vi "UHR-Fleezers Control (host) - 12.6.1.vi"() -> ()   [LabVIEW 2012] (continued)
        n1578 = Decrement(x=w2209) -> (x-1=w2210:u64)
        n1579 = Select(t=w2209, s=w2211, f=w2210) -> (s? t:f=w2208:u64)
        "Cycles/step (AOD)" <- w2208
        n1580 = xnode "Read/Write Control"("FPGA VI Reference In"=w2301, "error in"=w2300, "Scan steps"=w2240, "Number of scans"="Number of F/B Scans (AOD)", "Cycles per step"=w2208, "Scan freq.  increment"=w2246, "Scan BD"="Scan BD") -> ("error out"=w2299:errorcluster)  [unwired: 1 out]
        n1581 = Multiply(x=w2240, y=w2208) -> (x*y=w2294:u64)
        n1582 = Multiply(x=w2294, y=u64 2) -> (x*y=w2216:u64)
        n1583 = Multiply(x=w2217, y=w2216) -> (x*y=w2215:dbl)
        "Data points/scan (f/b)" <- w2215
        n1584 = Multiply(x=w2215, y="Number of F/B Scans (AOD)") -> (x*y=w2297:dbl)
        "Data points/scans" <- w2297
        n1585 = Divide(x=w2297, y=w2251) -> (x/y=→"N sets should be saved":dbl)
        n1586 = Multiply(x=w2294, y=w2235) -> (x*y=w2233:dbl)
        "Time/Scan (s) (AOD)" <- w2233
        n1587 = Select(t=w2265, s="Scan BD", f=0.0) -> (s? t:f=w2291:dbl)
        n1588 = Select(t=0.0, s="Scan BD", f=w2265) -> (s? t:f=w2287:dbl)
        n1589 = local read "BD 2 Frequency 2 (MHz)"() -> (w2283:dbl)
        n1590 = local read "BD 1 Frequency 2 (MHz)"() -> (w2286:dbl)
        n1591 = Add(x=w2287, y=w2258) -> (x+y=w2284:dbl)
        n1592 = Add(x=w2252, y=w2291) -> (x+y=w2285:dbl)
        n1593 = Multiply(x=w2233, y=2.0) -> (x*y=w2232:dbl)
        n1594 = Multiply(x=w2232, y="Number of F/B Scans (AOD)") -> (x*y=w2229:dbl)
        n1595 = Divide(x=w2229, y=60.0) -> (x/y=→"Time to Finish All (min)":dbl)
        n1596 = Add(x="Trap 2 Bead Size (nm)", y="Trap 1 Bead Size (nm)") -> (x+y=w2273:dbl)
        n1597 = Divide(x=w2273, y=2.0) -> (x/y=w2267:dbl)
        n1598 = local read "Initial delta (MHz)"() -> (w2270:dbl)
        n1599 = Subtract(x=w2284, y=w2283) -> (x-y=w2281:dbl)
        n1600 = Subtract(x=w2285, y=w2286) -> (x-y=w2282:dbl)
        n1601 = Square(x=w2281) -> (x^2=w2280:dbl)
        n1602 = Square(x=w2282) -> (x^2=w2279:dbl)
        n1603 = Add(x=w2279, y=w2280) -> (x+y=w2278:dbl)
        n1604 = Square Root(x=w2278) -> (sqrt(x)=w2277:dbl)
        "Final delta (MHz)" <- w2277
        n1605 = Multiply(x=w2269, y=w2277) -> (x*y=w2276:dbl)
        n1606 = Multiply(x=w2270, y=w2269) -> (x*y=w2268:dbl)
        n1607 = Subtract(x=w2268, y=w2267) -> (x-y=→"Initial sep (nm)":dbl)
        n1608 = Subtract(x=w2276, y=w2267) -> (x-y=→"Final sep (nm)":dbl)
      }
      event "Freq or Amp switch first", "Swap F1 and F2", "Freq switch delay", "Amp switch delay": Value Change {
        n1609 = event-data() -> ()  [unwired: 7 out]
        n1610 = local read "Amp switch delay"() -> (w2302:u16)
        n1611 = local read "Swap F1 and F2"() -> (w2303:bool)
        n1612 = xnode "Read/Write Control"("FPGA VI Reference In"=w2306, "error in"=w2305, "Swap F1 and F2"=w2303, "Amp switch delay"=w2302) -> ("error out"=w2304:errorcluster)  [unwired: 1 out]
      }
      event "Scan steps (MCL)", "Number of scans (MCL)", "Scan Range (V)\n(of steps)", "2D or 1D Scan", "N APD Samp/step", "Fast Scan Dir", "Continuous MCL Scanning", "Scan lines (y)": Value Change {
        w2308 = 32767.0 ("y")
        n1613 = event-data() -> ()  [unwired: 7 out]
        n1614 = Select(t="Scan lines (y)", s="2D or 1D Scan", f="Number of scans (MCL)") -> (s? t:f=w2313:u64)
        n1615 = Decrement(x="Scan steps (MCL)") -> (x-1=w2329:u64)
        n1616 = Divide(x="Scan Range (V)\n(of steps)", y=w2329) -> (x/y=w2328:dbl)
        "Desired Scan Incr (V)" <- w2328
        n1617 = local read "APD Integration Time (s)"() -> (w2321:dbl)
        n1618 = Multiply(x=w2328, y=w2308) -> (x*y=w2337:dbl)
        n1619 = Divide(x=w2337, y=10.0) -> (x/y=w2327:dbl)
        "Desired incr (int)" <- w2327
        n1620 = local read "Update Count (MCL)"() -> (w2333:u32)
        n1621 = Round Toward -Infinity(1:w2327) -> (0:w2336:dbl)
        n1622 = To Word Integer(number=w2336) -> (16bit integer=w2311:i16)
        "Actual Incr. int (MCL)" <- w2311
        n1623 = Multiply(x=w2321, y=40000000.0) -> (x*y=w2334:dbl)
        n1624 = Divide(x=w2334, y=w2333) -> (x/y=w2332:dbl)
        n1625 = Multiply(x=i16 10, y=w2311) -> (x*y=w2309:i16)
        n1626 = Multiply(x="N APD Samp/step", y=w2332) -> (x*y=w2331:dbl)
        "Cycles/step (MCL)" <- w2331
        n1627 = Divide(x=w2309, y=w2308) -> (x/y=→"Actual MCL Inc (V)":dbl)
        n1628 = Multiply(x="N APD Samp/step", y="Scan steps (MCL)") -> (x*y=w2323:dbl)
        n1629 = local read "APD Samples/FIFO Acq."() -> (w2320:dbl)
        n1630 = Multiply(x=w2323, y=u64 2) -> (x*y=w2322:dbl)
        "Data points/scan (f+b)" <- w2322
        n1631 = Multiply(x=w2322, y=w2313) -> (x*y=w2340:dbl)
        "Data points/scans (MCL)" <- w2340
        n1632 = Multiply(x=w2321, y=w2322) -> (x*y=w2314:dbl)
        "Time/f+b scan (s) (MCL)" <- w2314
        n1633 = Divide(x=w2340, y=w2320) -> (x/y=→"N sets should be saved (MCL)":dbl)
        n1634 = Multiply(x=w2314, y=w2313) -> (x*y=→"Total Time (s)":dbl)
        n1635 = Not(x="Fast Scan Dir") -> (.not. x?=w2318:bool)
        n1636 = xnode "Read/Write Control"("FPGA VI Reference In"=w2344, "error in"=w2343, "Scan steps (MCL)"="Scan steps (MCL)", "Number of scans (MCL)"=w2313, "Cycles per step (MCL)"=w2331, "Scan freq.  increment (MCL)"=w2311, "1D or 2D Scan?"="2D or 1D Scan", "MCL Scan Axis"=w2318, "Cont. Scan (MCL)"="Continuous MCL Scanning") -> ("error out"=w2342:errorcluster)  [unwired: 1 out]
      }
      event "Read Cal": Value Change {
        w2346 = 1000.0 ("y")
        n1637 = event-data() -> ()  [unwired: 7 out]
        n1638 = local read "Save file name"() -> (w2371:path)
        n1639 = local write "Read Cal"(FALSE ("Read Cal")) -> ()
        n1640 = Strip Path(path=w2371) -> (stripped path=w2370:path)  [unwired: 1 out]
        n1641 = Path To String(path=w2370) -> (string=w2369:string)
        n1642 = Concatenate Strings(w2369, "\\current.cal" ("string")) -> (w2367:string)
        n1643 = String To Path(string=w2367) -> (path=w2366:path)
        n1644 = Open/Create/Replace File(file path (use dialog)=w2366, operation (0:open)=T29."open", access (0:read/write)=enum16{"read/write", "read-only", "write-only"}."read-only") -> (refnum out=w2374:refnum<file>, error out=w2360:errorcluster)  [unwired: 1 in, 3 out]
        n1645 = Deny Access(4:w2360, 7:w2374) -> (0:w2359:errorcluster, 3:w2365:refnum<file>)  [unwired: 1 out]
        n1646 = Read from Binary File(5:0.0, 8:w2359, 9:T28."big-endian, network order" ("byte order (0:big-endian, network order)"), 10:-1 ("count (1)"), 11:w2365) -> (0:w2358:errorcluster, 2:w2356:dbl[], 3:w2361:refnum<file>)  [unwired: 2 out]
        n1647 = Array To Cluster(array=w2356) -> (cluster=w2355:T31)
        n1648 = Unbundle(w2355) -> ("[0]"=w2354:dbl, "[1]"=w2353:dbl, "[2]"=w2352:dbl, "[3]"=w2351:dbl, "[4]"=w2350:dbl, "[5]"=w2349:dbl)
        n1649 = Close File(refnum=w2361, error in=w2358) -> (error out=→"Read cal error":errorcluster)  [unwired: 1 out]
        n1650 = Multiply(x=w2349, y=w2346) -> (x*y=w2347:dbl)
        n1651 = local write "T2 kappa_x (pN/nm)"(w2351) -> ()
        n1652 = local write "T1 kappa_x (pN/nm)"(w2352) -> ()
        n1653 = local write "T1 alpha_x (nm/V)"(w2354) -> ()
        n1654 = local write "T2 alpha_x (nm/V)"(w2353) -> ()
        n1655 = Multiply(x=w2350, y=w2346) -> (x*y=w2348:dbl)
        n1656 = local write "T1 offset_x (mV)"(w2348) -> ()
        n1657 = local write "T2 offset_x (mV)"(w2347) -> ()
      }
      event "Abort MCL Scan": Value Change {
        n1658 = event-data() -> ()  [unwired: 7 out]
        n1659 = local write "MCL Scanning"(FALSE ("MCL Scanning")) -> ()
        n1660 = xnode "Read/Write Control"("FPGA VI Reference In"=w2379, "error in"=w2378, "Abort scan (MCL)"="Abort MCL Scan") -> ("error out"=w2377:errorcluster)  [unwired: 1 out]
      }
      event "Update Count (MCL)": Value Change {
        n1661 = event-data() -> ()  [unwired: 7 out]
        n1662 = xnode "Read/Write Control"("FPGA VI Reference In"=w2383, "error in"=w2382, "MCL count"="Update Count (MCL)") -> ("error out"=w2381:errorcluster)  [unwired: 1 out]
      }
      event "+ phase (MCL)", "- phase (MCL)": Value Change {
        n1663 = event-data() -> ()  [unwired: 7 out]
        n1664 = Or(x="- phase (MCL)", y="+ phase (MCL)") -> (x .or. y?=w2386:bool)
        n1665 = Negate(x="Phase adjust (MCL)") -> (-x=w2392:i16)
        n1666 = Select(t=w2392, s="+ phase (MCL)", f="Phase adjust (MCL)") -> (s? t:f=w2390:i16)
        n1667 = xnode "Read/Write Control"("FPGA VI Reference In"=w2394, "error in"=w2393, "Phase count adjustment (MCL)"=w2390) -> ("FPGA VI Reference Out"=w2387:T20, "error out"=w2388:errorcluster)
        n1668 = xnode "Read/Write Control"("FPGA VI Reference In"=w2387, "error in"=w2388, "+ phase (MCL)"=w2386) -> ("error out"=w2385:errorcluster)  [unwired: 1 out]
      }
      event "Abort AOD Scan": Value Change {
        n1669 = event-data() -> ()  [unwired: 7 out]
        n1670 = xnode "Read/Write Control"("FPGA VI Reference In"=w2398, "error in"=w2397, "Abort scan"="Abort AOD Scan") -> ("error out"=w2396:errorcluster)  [unwired: 1 out]
      }
      event "Continuous AOD Scanning": Value Change {
        n1671 = event-data() -> ()  [unwired: 7 out]
        n1672 = xnode "Read/Write Control"("FPGA VI Reference In"=w2402, "error in"=w2401, "Cont. Scan"="Continuous AOD Scanning") -> ("error out"=w2400:errorcluster)  [unwired: 1 out]
      }
      event "Index": Value Change {
        n1673 = event-data() -> ()  [unwired: 7 out]
        n1674 = call "Create new save file.vi"("Insert"="", "Ext"=".dat" ("string"), "Index In"="Index") -> ("Path Out"=→"Save file name":path, "Index Out"=w2403:dbl)
        "Save index" <- w2403
        n1675 = local write "Index"(w2403) -> ()
      }
      event "AO1", "AO2": Value Change {
        w2418 = 10.0 ("y")
        w2417 = 32767.0 ("y")
        n1676 = event-data() -> ()  [unwired: 7 out]
        n1677 = local read "AO2"() -> (w2416:dbl)
        n1678 = local read "AO1"() -> (w2413:dbl)
        n1679 = Multiply(x=w2413, y=w2417) -> (x*y=w2412:dbl)
        n1680 = Multiply(x=w2416, y=w2417) -> (x*y=w2415:dbl)
        n1681 = Divide(x=w2412, y=w2418) -> (x/y=w2411:dbl)
        n1682 = Divide(x=w2415, y=w2418) -> (x/y=w2414:dbl)
        n1683 = To Word Integer(number=w2411) -> (16bit integer=w2419:i16)
        n1684 = To Word Integer(number=w2414) -> (16bit integer=w2420:i16)
        n1685 = xnode "Read/Write Control"("FPGA VI Reference In"=w2410, "error in"=w2409, "AO1"=w2419, "AO2"=w2420) -> ("error out"=w2408:errorcluster)  [unwired: 1 out]
      }
      event "Inject Pump 1": Value Change {
        n1686 = event-data() -> ()  [unwired: 7 out]
        n1687 = local read "Use Harvard pumps\nfor beads (else Chemyx)"() -> (w2422:bool)
        n1688 = case shown="True" w2422 {
          tunnel: "Inject Pump 1" -> [w2426 w2464]
          tunnel: w2421 -> [_ w2465]
          frame False {
            n1689 = local read "Pump write delay (ms)"() -> (w2425:dbl)
            n1690 = local read "Chemyx Syringe Pump Serial Port"() -> (w2424:refnum<visa-resource-name>)
            n1691 = case shown="True" w2426 {
              tunnel: w2425 -> [w2432 w2446]
              tunnel: w2424 -> [w2429 w2445]
              frame False {
                n1692 = flat-sequence {
                  tunnel: w2429 -> [w2433]
                  tunnel: [w2433] -> w2430
                  tunnel: w2432 -> [_]
                  tunnel: [w2436] -> w2431
                  tunnel: w2430 -> [w2436]
                  tunnel: w2431 -> [w2437]
                  tunnel: [w2437] -> w2427
                  tunnel: [w2439] -> w2428
                  tunnel: w2427 -> [w2439]
                  tunnel: w2428 -> [w2441]
                  frame #0 {
                    n1693 = call "Write to pump.vi"("string"="enter pump1", "VISA resource name"=w2433) -> ()  [unwired: 1 out]
                  }
                  frame #1 {
                    n1694 = Wait (ms)(milliseconds to wait="Pump pause delay (ms)") -> ()  [unwired: 1 out]
                  }
                  frame #2 {
                    n1695 = call "Write to pump.vi"("string"="stop", "VISA resource name"=w2437) -> ()  [unwired: 1 out]
                  }
                  frame #3 {
                    n1696 = Wait (ms)(milliseconds to wait=u32 500) -> ()  [unwired: 1 out]
                  }
                  frame #4 {
                    n1697 = call "Write to pump.vi"("string"="stop", "VISA resource name"=w2441) -> ()  [unwired: 1 out]
                  }
                }
              }
              frame True {
                n1698 = flat-sequence {
                  tunnel: w2445 -> [w2455]
                  tunnel: w2446 -> [w2450]
                  tunnel: w2446 -> [w2457]
                  tunnel: w2445 -> [w2458]
                  tunnel: [w2458] -> w2443
                  tunnel: [w2460] -> w2444
                  tunnel: w2443 -> [w2460]
                  tunnel: w2444 -> [w2462]
                  frame #0 {
                    n1699 = local read "All Pump Parameters"() -> (w2449:T5)
                    n1700 = Unbundle By Name(w2449) -> ("Pump 1"=w2456:T32)
                    n1701 = call "Set pump parameters.vi"("Pump write delay (ms)"=w2450, "Volume (uL)"="Ch 1 Inject Volume (uL)", "Rate (uL/h)"="Ch 1 Inject Rate (ul/h)", "Units"=4.0, "Pump #"=1.0, "Pump Parameters In"=w2456, "VISA resource name"=w2455) -> ("Pump Parameters Out"=w2448:T32)  [unwired: 3 in]
                    n1702 = Bundle By Name(cluster=w2449, "Pump 1"=w2448) -> (w2447:T5)
                    n1703 = local write "All Pump Parameters"(w2447) -> ()
                  }
                  frame #1 {
                    n1704 = Wait (ms)(milliseconds to wait=w2457) -> ()  [unwired: 1 out]
                  }
                  frame #2 {
                    n1705 = call "Write to pump.vi"("string"="start", "VISA resource name"=w2458) -> ()  [unwired: 1 out]
                  }
                  frame #3 {
                    n1706 = Wait (ms)(milliseconds to wait=u32 500) -> ()  [unwired: 1 out]
                  }
                  frame #4 {
                    n1707 = call "Write to pump.vi"("string"="start", "VISA resource name"=w2462) -> ()  [unwired: 1 out]
                  }
                }
              }
            }
          }
          frame True {
            n1708 = case shown="False" w2464 {
              tunnel: w2465 -> [w2466 w2476]
              frame False {
                n1709 = flat-sequence {
                  tunnel: w2466 -> [w2468]
                  frame #0 {
                    n1710 = local write "Flushing P1"(FALSE ("Flushing P1")) -> ()
                    n1711 = Concatenate Strings("stop" ("string"), "\r") -> (w2470:string)
                    n1712 = VISA Write(VISA resource name=w2468, write buffer=w2470) -> ()  [unwired: 1 in, 3 out]
                  }
                  frame #1 {
                    n1713 = property on="Clear Volume P1" class="Bool (strict)"("Val(Sgnl)"=TRUE ("Value (Signaling)")) -> ()  [unwired: 2 in, 2 out]
                  }
                }
              }
              frame True {
                n1714 = local read "Normal Flow Rate (ul/h) P1"() -> (w2474:dbl)
                n1715 = Number To Decimal String(number=w2474) -> (decimal integer string=w2480:string)  [unwired: 1 in]
                n1716 = Concatenate Strings("irate  " ("string"), w2480, " u/h" ("string"), "\r") -> (w2478:string)
                n1717 = VISA Write(VISA resource name=w2476, write buffer=w2478) -> (VISA resource name out=w2475:refnum<visa-resource-name>)  [unwired: 1 in, 2 out]
                n1718 = Concatenate Strings("irun" ("string"), "\r") -> (w2482:string)
                n1719 = VISA Write(VISA resource name=w2475, write buffer=w2482) -> ()  [unwired: 1 in, 3 out]
              }
            }
          }
        }
      }
      event "Inject Pump 3": Value Change {
        n1720 = event-data() -> ()  [unwired: 7 out]
        n1721 = local read "Use Harvard pumps\nfor beads (else Chemyx)"() -> (w2485:bool)
        n1722 = case shown="True" w2485 {
          tunnel: "Inject Pump 3" -> [w2489 w2528]
          tunnel: w2484 -> [_ w2527]
          frame False {
            n1723 = local read "Pump write delay (ms)"() -> (w2488:dbl)
            n1724 = case shown="True" w2489 {
              tunnel: w2488 -> [w2495 w2509]
              tunnel: "Chemyx Syringe Pump Serial Port" -> [w2492 w2508]
              frame False {
                n1725 = flat-sequence {
                  tunnel: w2492 -> [w2496]
                  tunnel: [w2496] -> w2493
                  tunnel: w2495 -> [_]
                  tunnel: [w2499] -> w2494
                  tunnel: w2493 -> [w2499]
                  tunnel: w2494 -> [w2500]
                  tunnel: [w2500] -> w2490
                  tunnel: [w2502] -> w2491
                  tunnel: w2490 -> [w2502]
                  tunnel: w2491 -> [w2504]
                  frame #0 {
                    n1726 = call "Write to pump.vi"("string"="enter pump3", "VISA resource name"=w2496) -> ()  [unwired: 1 out]
                  }
                  frame #1 {
                    n1727 = local read "Pump pause delay (ms)"() -> (w2498:u32)
                    n1728 = Wait (ms)(milliseconds to wait=w2498) -> ()  [unwired: 1 out]
                  }
                  frame #2 {
                    n1729 = call "Write to pump.vi"("string"="stop", "VISA resource name"=w2500) -> ()  [unwired: 1 out]
                  }
                  frame #3 {
                    n1730 = Wait (ms)(milliseconds to wait=u32 0) -> ()  [unwired: 1 out]
                  }
                  frame #4 {
                    n1731 = call "Write to pump.vi"("string"="stop", "VISA resource name"=w2504) -> ()  [unwired: 1 out]
                  }
                }
              }
              frame True {
                n1732 = flat-sequence {
                  tunnel: w2508 -> [w2518]
                  tunnel: w2509 -> [w2513]
                  tunnel: w2509 -> [w2520]
                  tunnel: w2508 -> [w2521]
                  tunnel: [w2521] -> w2507
                  tunnel: [w2524] -> w2506
                  tunnel: w2507 -> [w2524]
                  tunnel: w2506 -> [w2525]
                  frame #0 {
                    n1733 = local read "All Pump Parameters"() -> (w2512:T5)
                    n1734 = Unbundle By Name(w2512) -> ("Pump 3"=w2519:T32)
                    n1735 = call "Set pump parameters.vi"("Pump write delay (ms)"=w2513, "Volume (uL)"="Ch 3 Inject Volume (uL)", "Rate (uL/h)"="Ch 3 Inject Rate (ul/h)", "Units"=4.0, "Pump #"=3.0, "Pump Parameters In"=w2519, "VISA resource name"=w2518) -> ("Pump Parameters Out"=w2511:T32)  [unwired: 3 in]
                    n1736 = Bundle By Name(cluster=w2512, "Pump 3"=w2511) -> (w2510:T5)
                    n1737 = local write "All Pump Parameters"(w2510) -> ()
                  }
                  frame #1 {
                    n1738 = Wait (ms)(milliseconds to wait=w2520) -> ()  [unwired: 1 out]
                  }
                  frame #2 {
                    n1739 = call "Write to pump.vi"("string"="start", "VISA resource name"=w2521) -> ()  [unwired: 1 out]
                  }
                  frame #3 {
                    n1740 = Wait (ms)(milliseconds to wait=u32 500) -> ()  [unwired: 1 out]
                  }
                  frame #4 {
                    n1741 = call "Write to pump.vi"("string"="start", "VISA resource name"=w2525) -> ()  [unwired: 1 out]
                  }
                }
              }
            }
          }
          frame True {
            n1742 = case shown="False" w2528 {
              tunnel: w2527 -> [w2529 w2536]
              frame False {
                n1743 = flat-sequence {
                  tunnel: w2529 -> [w2531]
                  frame #0 {
                    n1744 = local write "Flushing P3"(FALSE ("Flushing P3")) -> ()
                    n1745 = Concatenate Strings("stop" ("string"), "\r") -> (w2533:string)
                    n1746 = VISA Write(VISA resource name=w2531, write buffer=w2533) -> ()  [unwired: 1 in, 3 out]
                  }
                  frame #1 {
                    n1747 = property on="Clear Volume P3" class="Bool (strict)"("Val(Sgnl)"=TRUE ("Value (Signaling)")) -> ()  [unwired: 2 in, 2 out]
                  }
                }
              }
              frame True {
                n1748 = local read "Normal Flow Rate (ul/h) P3"() -> (w2537:dbl)
                n1749 = Number To Decimal String(number=w2537) -> (decimal integer string=w2543:string)  [unwired: 1 in]
                n1750 = Concatenate Strings("irate  " ("string"), w2543, " u/h" ("string"), "\r") -> (w2541:string)
                n1751 = VISA Write(VISA resource name=w2536, write buffer=w2541) -> (VISA resource name out=w2539:refnum<visa-resource-name>)  [unwired: 1 in, 2 out]
                n1752 = Concatenate Strings("irun" ("string"), "\r") -> (w2545:string)
                n1753 = VISA Write(VISA resource name=w2539, write buffer=w2545) -> ()  [unwired: 1 in, 3 out]
              }
            }
          }
        }
      }
      event "Inject Pump 2": Value Change {
        n1754 = event-data() -> ()  [unwired: 7 out]
        n1755 = local read "Pump write delay (ms)"() -> (w2549:dbl)
        n1756 = flat-sequence {
          tunnel: w2547 -> [w2562]
          tunnel: w2549 -> [w2558]
          tunnel: "Inject Pump 2" -> [_]
          tunnel: w2549 -> [w2564]
          tunnel: w2547 -> [w2565]
          frame #0 {
            n1757 = local read "All Pump Parameters"() -> (w2557:T5)
            n1758 = Multiply(x=60.0, y="Flush Center Ch Rate (ul/m)") -> (x*y=w2554:dbl)
            n1759 = Unbundle By Name(w2557) -> ("Pump 2"=w2563:T32)
            n1760 = call "Set pump parameters.vi"("Pump write delay (ms)"=w2558, "Volume (uL)"="Flush Center Ch Volume (uL)", "Rate (uL/h)"=w2554, "Units"=3.0, "Pump #"=2.0, "Pump Parameters In"=w2563, "VISA resource name"=w2562) -> ("Pump Parameters Out"=w2556:T32)  [unwired: 3 in]
            n1761 = Bundle By Name(cluster=w2557, "Pump 2"=w2556) -> (w2555:T5)
            n1762 = local write "All Pump Parameters"(w2555) -> ()
            n1763 = Add(x="Flush Center Ch Volume (uL)", y="Total Volume\nFlushed (uL)") -> (x+y=w2551:dbl)
            n1764 = local write "Total Volume\nFlushed (uL)"(w2551) -> ()
          }
          frame #1 {
            n1765 = Wait (ms)(milliseconds to wait=w2564) -> ()  [unwired: 1 out]
          }
          frame #2 {
            n1766 = call "Write to pump.vi"("string"="start", "VISA resource name"=w2565) -> ()  [unwired: 1 out]
          }
        }
        n1767 = local read "Chemyx Syringe Pump Serial Port"() -> (w2547:refnum<visa-resource-name>)
      }
      event "Sample Channel\nFlow": Value Change {
        n1768 = event-data() -> ()  [unwired: 7 out]
        n1769 = Select(t="irun" ("string"), s="Sample Channel\nFlow", f="stop" ("string")) -> (s? t:f=w2569:string)
        n1770 = Concatenate Strings(w2569, "\r") -> (w2572:string)
        n1771 = VISA Write(VISA resource name=w2567, write buffer=w2572) -> ()  [unwired: 1 in, 3 out]
      }
      event "Start Flow": Value Change {
        n1772 = event-data() -> ()  [unwired: 7 out]
        n1773 = local write "Sample Channel\nFlow"(TRUE ("Sample Channel\nFlow")) -> ()
        n1774 = local write "Start Flow"(FALSE ("Start Flow")) -> ()
        n1775 = Concatenate Strings("irun" ("string"), "\r") -> (w2578:string)
        n1776 = VISA Write(VISA resource name=w2574, write buffer=w2578) -> ()  [unwired: 1 in, 3 out]
      }
      event "Stop Flow": Value Change {
        w2580 = FALSE ("Stop Flow")
        n1777 = event-data() -> ()  [unwired: 7 out]
        n1778 = local write "Stop Flow"(w2580) -> ()
        n1779 = local write "Sample Channel\nFlow"(w2580) -> ()
        n1780 = Concatenate Strings("stop" ("string"), "\r") -> (w2583:string)
        n1781 = VISA Write(VISA resource name=w2581, write buffer=w2583) -> ()  [unwired: 1 in, 3 out]
      }
      event "Flow rate (uL/h)": Value Change {
        n1782 = event-data() -> ()  [unwired: 7 out]
        n1783 = Number To Decimal String(number="Flow rate (uL/h)") -> (decimal integer string=w2590:string)  [unwired: 1 in]
        n1784 = Concatenate Strings("irate  " ("string"), w2590, " u/h" ("string"), "\r") -> (w2589:string)
        n1785 = VISA Write(VISA resource name=w2586, write buffer=w2589) -> ()  [unwired: 1 in, 3 out]
      }
      event "Flush Sample": Value Change {
        n1786 = event-data() -> ()  [unwired: 7 out]
        n1787 = flat-sequence {
          tunnel: w2595 -> [w2623]
          tunnel: [w2603] -> w2594
          tunnel: [w2597] -> w2592
          tunnel: w2594 -> [w2627]
          tunnel: [w2627] -> w2593
          tunnel: w2592 -> [w2626]
          tunnel: w2593 -> [w2632]
          frame #0 {
            # "set paramaters (rate, volume) for flush, clear volume"
            n1788 = Number To Decimal String(number="Flush rate (uL/m)") -> (decimal integer string=w2619:string)  [unwired: 1 in]
            n1789 = Concatenate Strings("irate  " ("string"), w2619, " u/m" ("string"), "\r") -> (w2621:string)
            n1790 = VISA Write(VISA resource name=w2623, write buffer=w2621) -> (VISA resource name out=w2617:refnum<visa-resource-name>)  [unwired: 1 in, 2 out]
            n1791 = Reciprocal(x="Flush rate (uL/m)") -> (1/x=w2600:dbl)
            n1792 = Number To Decimal String(number="Volume (uL)") -> (decimal integer string=w2608:string)  [unwired: 1 in]
            n1793 = Multiply(x="Volume (uL)", y=w2600) -> (x*y=w2599:dbl)
            n1794 = Concatenate Strings("tvolume  " ("string"), w2608, " u" ("string"), "\r") -> (w2606:string)
            n1795 = Multiply(x=w2599, y=60000.0) -> (x*y=w2597:dbl)
            n1796 = VISA Write(VISA resource name=w2617, write buffer=w2606) -> (VISA resource name out=w2605:refnum<visa-resource-name>)  [unwired: 1 in, 2 out]
            n1797 = Concatenate Strings("cvolume" ("string"), "\r") -> (w2604:string)
            n1798 = VISA Write(VISA resource name=w2605, write buffer=w2604) -> (VISA resource name out=w2615:refnum<visa-resource-name>)  [unwired: 1 in, 2 out]
            n1799 = Concatenate Strings("irun" ("string"), "\r") -> (w2613:string)
            n1800 = VISA Write(VISA resource name=w2615, write buffer=w2613) -> (VISA resource name out=w2603:refnum<visa-resource-name>)  [unwired: 1 in, 2 out]
          }
          frame #1 {
            # "Have to wait until\nflow is done to reset\nrate"
            n1801 = Add(x=w2626, y=100.0) -> (x+y=w2625:dbl)
            n1802 = Wait (ms)(milliseconds to wait=w2625) -> ()  [unwired: 1 out]
          }
          frame #2 {
            # "reset flow rate to usual flow rate"
            n1803 = local read "Flow rate (uL/h)"() -> (w2638:dbl)
            n1804 = Number To Decimal String(number=w2638) -> (decimal integer string=w2636:string)  [unwired: 1 in]
            n1805 = Concatenate Strings("irate  " ("string"), w2636, " u/h" ("string"), "\r") -> (w2634:string)
            n1806 = VISA Write(VISA resource name=w2632, write buffer=w2634) -> (VISA resource name out=w2628:refnum<visa-resource-name>)  [unwired: 1 in, 2 out]
            n1807 = Concatenate Strings("cvolume" ("string"), "\r") -> (w2629:string)
            n1808 = VISA Write(VISA resource name=w2628, write buffer=w2629) -> ()  [unwired: 1 in, 3 out]
          }
        }
      }
      event "Flush Pump 3": Value Change {
        n1809 = event-data() -> ()  [unwired: 7 out]
        n1810 = flat-sequence {
          tunnel: w2639 -> [w2642]
          frame #0 {
            # "set paramaters (rate, volume) for flush, clear volume"
            n1811 = Number To Decimal String(number="Flush rate (uL/m) P3") -> (decimal integer string=w2664:string)  [unwired: 1 in]
            n1812 = local write "Inject Pump 3"(TRUE ("Inject Pump 3")) -> ()
            n1813 = Concatenate Strings("irate  " ("string"), w2664, " u/m" ("string"), "\r") -> (w2666:string)
            n1814 = VISA Write(VISA resource name=w2642, write buffer=w2666) -> (VISA resource name out=w2662:refnum<visa-resource-name>)  [unwired: 1 in, 2 out]
            n1815 = Reciprocal(x="Flush rate (uL/m) P3") -> (1/x=w2646:dbl)
            n1816 = Number To Decimal String(number="Volume (uL) P3") -> (decimal integer string=w2653:string)  [unwired: 1 in]
            n1817 = Multiply(x="Volume (uL) P3", y=w2646) -> (x*y=w2645:dbl)
            n1818 = Concatenate Strings("tvolume  " ("string"), w2653, " u" ("string"), "\r") -> (w2651:string)
            n1819 = Multiply(x=w2645, y=60.0) -> (x*y=→"HP3 Flush Time (s)":dbl)
            n1820 = VISA Write(VISA resource name=w2662, write buffer=w2651) -> (VISA resource name out=w2650:refnum<visa-resource-name>)  [unwired: 1 in, 2 out]
            n1821 = Concatenate Strings("cvolume" ("string"), "\r") -> (w2649:string)
            n1822 = VISA Write(VISA resource name=w2650, write buffer=w2649) -> (VISA resource name out=w2660:refnum<visa-resource-name>)  [unwired: 1 in, 2 out]
            n1823 = Concatenate Strings("irun" ("string"), "\r") -> (w2658:string)
            n1824 = VISA Write(VISA resource name=w2660, write buffer=w2658) -> ()  [unwired: 1 in, 3 out]
          }
          frame #1 {
            "Flushing P3" <- TRUE ("Flushing P3")
          }
        }
      }
      event "Flush Pump 1": Value Change {
        n1825 = event-data() -> ()  [unwired: 7 out]
        n1826 = flat-sequence {
          tunnel: [w2680] -> w2670
          tunnel: w2669 -> [w2673]
          tunnel: w2670 -> [_]
          frame #0 {
            # "set paramaters (rate, volume) for flush, clear volume"
            n1827 = local write "Inject Pump 1"(TRUE ("Inject Pump 1")) -> ()
            n1828 = Number To Decimal String(number="Flush rate (uL/m) P1") -> (decimal integer string=w2696:string)  [unwired: 1 in]
            n1829 = Concatenate Strings("irate  " ("string"), w2696, " u/m" ("string"), "\r") -> (w2698:string)
            n1830 = VISA Write(VISA resource name=w2673, write buffer=w2698) -> (VISA resource name out=w2694:refnum<visa-resource-name>)  [unwired: 1 in, 2 out]
            n1831 = Reciprocal(x="Flush rate (uL/m) P1") -> (1/x=w2677:dbl)
            n1832 = Number To Decimal String(number="Volume (uL) P1") -> (decimal integer string=w2685:string)  [unwired: 1 in]
            n1833 = Multiply(x="Volume (uL) P1", y=w2677) -> (x*y=w2676:dbl)
            n1834 = Concatenate Strings("tvolume  " ("string"), w2685, " u" ("string"), "\r") -> (w2683:string)
            n1835 = Multiply(x=w2676, y=60.0) -> (x*y=→"HP1 Flush Time (s)":dbl)
            n1836 = VISA Write(VISA resource name=w2694, write buffer=w2683) -> (VISA resource name out=w2682:refnum<visa-resource-name>)  [unwired: 1 in, 2 out]
            n1837 = Concatenate Strings("cvolume" ("string"), "\r") -> (w2681:string)
            n1838 = VISA Write(VISA resource name=w2682, write buffer=w2681) -> (VISA resource name out=w2692:refnum<visa-resource-name>)  [unwired: 1 in, 2 out]
            n1839 = Concatenate Strings("irun" ("string"), "\r") -> (w2690:string)
            n1840 = VISA Write(VISA resource name=w2692, write buffer=w2690) -> (VISA resource name out=w2680:refnum<visa-resource-name>)  [unwired: 1 in, 2 out]
          }
          frame #1 {
            "Flushing P1" <- TRUE ("Flushing P3")
          }
        }
      }
      event "Clear Volume": Value Change {
        n1841 = event-data() -> ()  [unwired: 7 out]
        n1842 = Concatenate Strings("cvolume" ("string"), "\r") -> (w2702:string)
        n1843 = VISA Write(VISA resource name=w2701, write buffer=w2702) -> ()  [unwired: 1 in, 3 out]
      }
      event "Clear Volume P3": Value Change {
        n1844 = event-data() -> ()  [unwired: 7 out]
        n1845 = Concatenate Strings("cvolume" ("string"), "\r") -> (w2708:string)
        n1846 = VISA Write(VISA resource name=w2707, write buffer=w2708) -> ()  [unwired: 1 in, 3 out]
        n1847 = local write "Clear Volume P3"(FALSE ("Clear Volume P3")) -> ()
      }
      event "Clear Volume P1": Value Change {
        n1848 = event-data() -> ()  [unwired: 7 out]
        n1849 = Concatenate Strings("cvolume" ("string"), "\r") -> (w2713:string)
        n1850 = local write "Clear Volume P1"(FALSE ("Clear Volume P1")) -> ()
        n1851 = VISA Write(VISA resource name=w2712, write buffer=w2713) -> ()  [unwired: 1 in, 3 out]
      }
      event "Display On P3": Value Change {
        n1852 = event-data() -> ()  [unwired: 7 out]
        n1853 = Select(t="dim 100", s="Display On P3", f="dim 0") -> (s? t:f=w2719:string)
        n1854 = Concatenate Strings(w2719, "\r") -> (w2721:string)
        n1855 = VISA Write(VISA resource name=w2716, write buffer=w2721) -> ()  [unwired: 1 in, 3 out]
      }
      event "Display On P1": Value Change {
        n1856 = event-data() -> ()  [unwired: 7 out]
        n1857 = Select(t="dim 100", s="Display On P1", f="dim 0") -> (s? t:f=w2726:string)
        n1858 = Concatenate Strings(w2726, "\r") -> (w2728:string)
        n1859 = VISA Write(VISA resource name=w2723, write buffer=w2728) -> ()  [unwired: 1 in, 3 out]
      }
      event "Retract Pump 3": Value Change {
        n1860 = event-data() -> ()  [unwired: 7 out]
        n1861 = local write "Retract Pump 3"(FALSE ("Retract Pump 3")) -> ()
        n1862 = case shown="True" "Retract Pump 3" {
          tunnel: w2730 -> [_ w2733]
          frame False {
          }
          frame True {
            n1863 = Number To Decimal String(number="Retract Rate (uL/m)") -> (decimal integer string=w2751:string)  [unwired: 1 in]
            n1864 = Concatenate Strings("wrate  " ("string"), w2751, " u/m" ("string"), "\r") -> (w2753:string)
            n1865 = VISA Write(VISA resource name=w2733, write buffer=w2753) -> (VISA resource name out=w2744:refnum<visa-resource-name>)  [unwired: 1 in, 2 out]
            n1866 = Number To Decimal String(number="Retract Vol 3 (uL)") -> (decimal integer string=w2746:string)  [unwired: 1 in]
            n1867 = Concatenate Strings("tvolume  " ("string"), w2746, " u" ("string"), "\r") -> (w2743:string)
            n1868 = VISA Write(VISA resource name=w2744, write buffer=w2743) -> (VISA resource name out=w2739:refnum<visa-resource-name>)  [unwired: 1 in, 2 out]
            n1869 = Concatenate Strings("cvolume" ("string"), "\r") -> (w2740:string)
            n1870 = VISA Write(VISA resource name=w2739, write buffer=w2740) -> (VISA resource name out=w2734:refnum<visa-resource-name>)  [unwired: 1 in, 2 out]
            n1871 = Concatenate Strings("wrun" ("string"), "\r") -> (w2735:string)
            n1872 = VISA Write(VISA resource name=w2734, write buffer=w2735) -> ()  [unwired: 1 in, 3 out]
          }
        }
      }
      event "Retract Pump 1": Value Change {
        n1873 = event-data() -> ()  [unwired: 7 out]
        n1874 = local write "Retract Pump 1"(FALSE ("Retract Pump 1")) -> ()
        n1875 = case shown="True" "Retract Pump 1" {
          tunnel: w2755 -> [_ w2760]
          frame False {
          }
          frame True {
            n1876 = local read "Retract Rate (uL/m)"() -> (w2758:dbl)
            n1877 = Number To Decimal String(number=w2758) -> (decimal integer string=w2776:string)  [unwired: 1 in]
            n1878 = Concatenate Strings("wrate  " ("string"), w2776, " u/m" ("string"), "\r") -> (w2778:string)
            n1879 = VISA Write(VISA resource name=w2760, write buffer=w2778) -> (VISA resource name out=w2770:refnum<visa-resource-name>)  [unwired: 1 in, 2 out]
            n1880 = Number To Decimal String(number="Retract Vol 1 (uL)") -> (decimal integer string=w2772:string)  [unwired: 1 in]
            n1881 = Concatenate Strings("tvolume  " ("string"), w2772, " u" ("string"), "\r") -> (w2769:string)
            n1882 = VISA Write(VISA resource name=w2770, write buffer=w2769) -> (VISA resource name out=w2766:refnum<visa-resource-name>)  [unwired: 1 in, 2 out]
            n1883 = Concatenate Strings("cvolume" ("string"), "\r") -> (w2767:string)
            n1884 = VISA Write(VISA resource name=w2766, write buffer=w2767) -> (VISA resource name out=w2761:refnum<visa-resource-name>)  [unwired: 1 in, 2 out]
            n1885 = Concatenate Strings("wrun" ("string"), "\r") -> (w2762:string)
            n1886 = VISA Write(VISA resource name=w2761, write buffer=w2762) -> ()  [unwired: 1 in, 3 out]
          }
        }
      }
      event "Flip Green Filter": Value Change {
        n1887 = event-data() -> ()  [unwired: 7 out]
        n1888 = Not(x="Flip Green Filter") -> (.not. x?=w2780:bool)
        n1889 = local write "Flip Green Filter"(w2780) -> ()
        n1890 = flat-sequence {
          tunnel: w2788 -> [w2793]
          tunnel: w2787 -> [w2792]
          tunnel: [w2790] -> w2785
          tunnel: [w2789] -> w2784
          tunnel: [w2795] -> w2783
          tunnel: w2785 -> [w2795]
          tunnel: [w2794] -> w2782
          tunnel: w2784 -> [w2794]
          tunnel: w2783 -> [w2799]
          tunnel: w2782 -> [w2798]
          tunnel: [w2797] -> w2786
          frame #0 {
            n1891 = xnode "Read/Write Control"("FPGA VI Reference In"=w2793, "error in"=w2792, "Green Filter Flipper"=TRUE) -> ("FPGA VI Reference Out"=w2790:T20, "error out"=w2789:errorcluster)
          }
          frame #1 {
            n1892 = Wait (ms)(milliseconds to wait=u32 100) -> ()  [unwired: 1 out]
          }
          frame #2 {
            n1893 = xnode "Read/Write Control"("FPGA VI Reference In"=w2799, "error in"=w2798, "Green Filter Flipper"=FALSE) -> ("error out"=w2797:errorcluster)  [unwired: 1 out]
          }
        }
      }
      event "Pump 1 contents", "Pump 3 contents": Value Change {
        n1894 = event-data() -> ()  [unwired: 7 out]
        n1895 = local read "Pump 1 contents"() -> (→"Pump 1 cont disp":string)
        n1896 = local read "Pump 3 contents"() -> (→"Pump 3 cont disp":string)
      }
      event "Reset Trap Pos. FB": Value Change {
        n1897 = event-data() -> ()  [unwired: 7 out]
        n1898 = xnode "Read/Write Control"("FPGA VI Reference In"=w2805, "error in"=w2804, "Trap Pos. FB Reset"="Reset Trap Pos. FB") -> ()  [unwired: 2 out]
      }
      event "Rem fb disp offset": Value Change {
        n1899 = event-data() -> ()  [unwired: 7 out]
        n1900 = local write "Rem fb disp offset"(FALSE ("Rem fb disp offset")) -> ()
        n1901 = local read "Mean T1 Position (nm)"() -> (w2807:dbl)
        n1902 = local read "FB Trap Pos Offset"() -> (w2808:dbl)
        n1903 = Subtract(x=w2808, y=w2807) -> (x-y=w2806:dbl)
        n1904 = local write "FB Trap Pos Offset"(w2806) -> ()
      }
      event "Threshold (nm)": Value Change {
        n1905 = event-data() -> ()  [unwired: 7 out]
        n1906 = flat-sequence {
          tunnel: w2812 -> [w2820]
          tunnel: w2811 -> [w2819]
          tunnel: [w2813] -> w2810
          tunnel: w2810 -> [w2826]
          frame #0 {
            n1907 = xnode "Read/Write Control"("FPGA VI Reference In"=w2820, "error in"=w2819) -> ("FPGA VI Reference Out"=w2816:T20, "error out"=w2815:errorcluster, "FPGA TTrig Thresh"=w2817:i64)
            n1908 = local read "Threshold stored (nm)"() -> (w2825:dbl)
            n1909 = local read "Threshold (nm)"() -> (w2813:dbl)
            n1910 = local read "AOM X Cal (nm/MHz)"() -> (w2823:dbl)
            n1911 = Subtract(x=w2813, y=w2825) -> (x-y=w2824:dbl)
            n1912 = Divide(x=w2824, y=w2823) -> (x/y=w2821:dbl)
            n1913 = call "IR AOM freq to word.vi"("Frequency In (MHz)"=w2821) -> ("Frequency Word Out (double)"=w2822:dbl)
            n1914 = To Quad Integer(1:w2822) -> (0:w2818:i64)
            n1915 = Add(x=w2817, y=w2818) -> (x+y=w2814:i64)
            n1916 = xnode "Read/Write Control"("FPGA VI Reference In"=w2816, "error in"=w2815, "FPGA TTrig Thresh"=w2814) -> ()  [unwired: 2 out]
          }
          frame #1 {
            "Threshold stored (nm)" <- w2826
          }
        }
      }
      event "FB Trig Integrate": Value Change {
        n1917 = event-data() -> ()  [unwired: 7 out]
        n1918 = local read "FB Trig Integrate"() -> (w2828:u32)
        n1919 = xnode "Read/Write Control"("FPGA VI Reference In"=w2830, "error in"=w2829, "FB Trig Integrate"=w2828) -> ("error out"=w2827:errorcluster)  [unwired: 1 out]
      }
      event "11": Value Change {
        n1920 = event-data() -> ()  [unwired: 7 out]
        n1921 = local read "11"() -> (w2831:bool)
        n1922 = case shown="True" w2831 {
          frame False {
          }
          frame True {
            n1923 = local read "Messages"() -> (w2833:string)
            n1924 = call "Update messages.vi"("Message to add"="You kicked it up to 11!", "Old message string"=w2833) -> ("New message string"=w2834:string)
            n1925 = call <vilib>:"Beep.vi"() -> ()  [unwired: 12 in]
            n1926 = local write "Messages"(w2834) -> ()
          }
        }
      }
      event "Trap Pos. FB ON": Value Change {
        n1927 = event-data() -> ()  [unwired: 7 out]
        n1928 = xnode "Read/Write Control"("FPGA VI Reference In"=w2837, "error in"=w2836, "Force feedback"="Trap Pos. FB ON") -> ()  [unwired: 2 out]
      }
      event "Remove Action Offset": Value Change {
        n1929 = event-data() -> ()  [unwired: 7 out]
        n1930 = local write "Remove Action Offset"(FALSE ("Remove Action Offset")) -> ()
        n1931 = local read "Trap Pos. FB Mult Factor"() -> (w2842:i64)
        n1932 = local read "Trap Pos FB Action"() -> (w2840:i64)
        n1933 = local read "Trap Pos. FB Offset Factor"() -> (w2838:i64)
        n1934 = Multiply(x=w2842, y=w2840) -> (x*y=w2841:i64)
        n1935 = Add(x=w2841, y=w2838) -> (x+y=w2839:i64)
        n1936 = local write "Trap Pos. FB Offset Factor"(w2839) -> ()
        n1937 = xnode "Read/Write Control"("FPGA VI Reference In"=w2845, "error in"=w2844, "Trap Pos. FB Offset Factor"=w2839) -> ()  [unwired: 2 out]
      }
      event "Remove Unwinding Offset": Value Change {
        n1938 = event-data() -> ()  [unwired: 7 out]
        n1939 = local write "Remove Unwinding Offset"(FALSE ("Remove Action Offset")) -> ()
        n1940 = local read "Trap Pos. FB Mult Factor"() -> (w2857:i64)
        n1941 = local read "Trap Pos FB Action"() -> (w2855:i64)
        n1942 = local read "Trap Pos. FB Offset Factor"() -> (w2854:i64)
        n1943 = Multiply(x=w2857, y=w2855) -> (x*y=w2856:i64)
        n1944 = local read "Trap Pos. FB Mult Factor"() -> (w2853:i64)
        n1945 = Add(x=w2856, y=w2854) -> (x+y=w2847:i64)
        n1946 = Multiply(x=32768, y="factor") -> (x*y=w2850:dbl)
        n1947 = Multiply(x=w2850, y=w2853) -> (x*y=w2852:dbl)
        n1948 = Subtract(x=w2847, y=w2852) -> (x-y=w2851:dbl)
        n1949 = To Quad Integer(1:w2851) -> (0:w2846:i64)
        n1950 = xnode "Read/Write Control"("FPGA VI Reference In"=w2860, "error in"=w2859, "Trap Pos. FB Offset Factor"=w2846) -> ()  [unwired: 2 out]
        n1951 = local write "Trap Pos. FB Offset Factor"(w2846) -> ()
      }
      event "Trap Pos. FB Range", "Trap Pos. FB Gains", "Trap Pos. FB Mult Factor", "Trap Pos. FB Offset Factor", "Trap Pos FB Negate Action", "Trap Pos FB Monitor\nT1 or T2", "Differential FB?", "Negate Diff?": Value Change {
        n1952 = event-data() -> ()  [unwired: 7 out]
        n1953 = Unbundle By Name("Trap Pos. FB Gains") -> ("proportional gain (Kc)"=w2863:fxp<+/-,16,8>, "integral gain (Kc*Ts/Ti)"=w2862:fxp<+/-,16,8>, "derivative gain (Kc*Td/Ts)"=w2861:fxp<+/-,16,8>)
        n1954 = local read "Negate Diff?"() -> (w2868:bool)
        n1955 = Unbundle By Name("Trap Pos. FB Range") -> ("output high"=w2866:fxp<+/-,16,1>, "output low"=w2865:fxp<+/-,16,1>)
        n1956 = xnode "Read/Write Control"("FPGA VI Reference In"=w2876, "error in"=w2875, "FB2 output high"=w2866, "FB2 output low"=w2865, "P2"=w2863, "I2"=w2862, "D2"=w2861, "Trap Pos. FB Mult Factor"="Trap Pos. FB Mult Factor", "Trap Pos. FB Offset Factor"="Trap Pos. FB Offset Factor", "Trap Pos FB Negate Action"="Trap Pos FB Negate Action", "Trap Pos FB Monitor T1 or T2"="Trap Pos FB Monitor\nT1 or T2", "AI1 X Scale"="Trap Pos. AI1 X Pre-scale", "Negate Diff?"=w2868, "Diff FB Measurement?"="Differential FB?") -> ()  [unwired: 2 out]
      }
      event "Trap Pos FB SP", "Trap Pos FB SP 2", "Use SP 2": Value Change {
        n1957 = event-data() -> ()  [unwired: 7 out]
        n1958 = Select(t="Trap Pos FB SP 2", s="Use SP 2", f="Trap Pos FB SP") -> (s? t:f=w2877:fxp<+/-,16,1>)
        n1959 = xnode "Read/Write Control"("FPGA VI Reference In"=w2882, "error in"=w2881, "Trap Pos. FB SP"=w2877) -> ()  [unwired: 2 out]
      }
      event "Offset SP2 from SP1": Value Change {
        n1960 = event-data() -> ()  [unwired: 7 out]
        n1961 = local read "Trap Pos FB SP"() -> (w2885:fxp<+/-,16,1>)
        n1962 = Add(x=w2885, y="SP2 Offset") -> (x+y=w2883:fxp<+/-,16,1>)
        n1963 = property on="Trap Pos FB SP 2" class="DigNum (strict)"("Val(Sgnl)"=w2883) -> ()  [unwired: 2 in, 2 out]
        n1964 = local write "Offset SP2 from SP1"(FALSE ("Offset SP2 from SP1")) -> ()
      }
      event "Set Reading to\nSetpoint": Value Change {
        # "This is the actual PID input signal"
        n1965 = event-data() -> ()  [unwired: 7 out]
        n1966 = local write "Set Reading to\nSetpoint"(FALSE ("Set SP to Reading")) -> ()
        n1967 = xnode "Read/Write Control"("FPGA VI Reference In"=w2891, "error in"=w2890) -> ("FPGA VI Reference Out"=w2889:T20, "error out"=w2888:errorcluster, "Trap Pos FB Int-Norm Signal"=w2887:fxp<+/-,16,1>)
        n1968 = local read "Differential FB?"() -> (w2892:bool)
        n1969 = case shown="False" w2892 {
          tunnel: [w2897 w2904] -> w2894
          tunnel: w2887 -> [w2895 w2904]
          frame False {
            n1970 = local read "Trap Pos FB Monitor\nT1 or T2"() -> (w2900:bool)
            n1971 = local read "Trap X AI1 (DMA)"() -> (w2903:T13)
            n1972 = Unbundle By Name(w2903) -> ("Set 1"=w2902:fxp<+/-,16,1>, "Set 2"=w2901:fxp<+/-,16,1>)
            n1973 = Select(t=w2902, s=w2900, f=w2901) -> (s? t:f=w2899:fxp<+/-,16,1>)
            n1974 = Not(x="Set SP Using...") -> (.not. x?=w2896:bool)
            n1975 = Select(t=w2895, s=w2896, f=w2899) -> (s? t:f=w2897:fxp<+/-,16,1>)
          }
          frame True {
          }
        }
        n1976 = xnode "Read/Write Control"("FPGA VI Reference In"=w2889, "error in"=w2888, "Trap Pos. FB SP"=w2894) -> ()  [unwired: 2 out]
        n1977 = local write "Trap Pos FB SP"(w2894) -> ()
      }
      event "Trap Pos. FB Out Scale 2^n": Value Change {
        n1978 = event-data() -> ()  [unwired: 7 out]
        n1979 = Scale By Power Of 2(n="Trap Pos. FB Out Scale 2^n", x=ext 1.0) -> (x*2^n=w2905:ext)
        n1980 = property on="Trap Pos. FB Mult Factor" class="DigNum (strict)"("Val(Sgnl)"=w2905) -> ()  [unwired: 2 in, 2 out]
      }
      event "Trap Pos FB Int Count": Value Change {
        n1981 = event-data() -> ()  [unwired: 7 out]
        n1982 = xnode "Read/Write Control"("FPGA VI Reference In"=w2910, "error in"=w2909, "Trap Pos FB Int Count"="Trap Pos FB Int Count") -> ()  [unwired: 2 out]
      }
      event "Trap pos": Value Change {
        n1983 = event-data() -> ()  [unwired: 7 out]
        n1984 = case shown="True" "Trap pos" {
          frame False {
            n1985 = property on="Trap Delta Graph" class="WFGraph (strict)"("Visible"=TRUE) -> ()  [unwired: 2 in, 2 out]
            n1986 = property on="Saved trap pos" class="WFGraph (strict)"("Visible"=FALSE) -> ()  [unwired: 2 in, 2 out]
          }
          frame True {
            n1987 = property on="Saved trap pos" class="WFGraph (strict)"("Visible"=TRUE) -> ()  [unwired: 2 in, 2 out]
            n1988 = property on="Trap Delta Graph" class="WFGraph (strict)"("Visible"=FALSE) -> ()  [unwired: 2 in, 2 out]
          }
        }
      }
    }
    "error out 2" <- w1733
    n1989 = node-c288() -> ()  [unwired: 2 out]
  }
  n1990 = while "Duncan's play event loop" {
    stop <- w2917 stop-if-true
    n1991 = Create User Event(user event datatype=TRUE ("Boolean")) -> (user event=w2918:refnum<user-event>)  [unwired: 1 in, 1 out]
    n1992 = Create User Event(user event datatype=TRUE ("Boolean")) -> (user event=w2925:refnum<user-event>)  [unwired: 1 in, 1 out]
    n1993 = global write "Global for fluorescence simulation mean (30 samples), (power series).vi" "Red Signal"(w2918) -> ()
    n1994 = global write "Global for fluorescence simulation mean (30 samples), (power series).vi" "Green Signal"(w2925) -> ()
    n1995 = register-events(w2925, w2918) -> (reference out=w2924:refnum<event-registration>)  [unwired: 2 in, 1 out]
    n1996 = event shown="[1] \"Get Fluorophore\": Value Change" {
      selector: w2924 -> [_ _ _ _]
      dyn-events: _ -> [_ _ _ _]
      timeout: 100 -> [_ _ _ _]
      event Timeout {
        n1997 = event-data() -> ()  [unwired: 1 in, 2 out]
      }
      event "Get Fluorophore": Value Change {
        n1998 = event-data() -> ("OldVal"=w2927:bool)  [unwired: 1 in, 4 out]
        n1999 = case shown="True" w2927 {
          selector: w2927 -> [_ w2928]
          frame False {
          }
          frame True {
            n2000 = property on="Move to Position 3" class="Bool"("Val(Sgnl)"=w2928) -> ()  [unwired: 2 in, 2 out]
            n2001 = case shown="1" "Numeric" {
              frame 0, Default {
              }
              frame 1 {
                n2002 = property on="Green Laser ON" class="Bool (strict)"("Val(Sgnl)"=TRUE ("Value (Signaling)")) -> ()  [unwired: 2 in, 2 out]
              }
              frame 2 {
                n2003 = property on="Red Laser ON" class="Bool (strict)"("Val(Sgnl)"=TRUE) -> ()  [unwired: 2 in, 2 out]
              }
            }
          }
        }
      }
      event User Event {
        n2004 = event-data() -> ("Boolean"=w2932:bool)  [unwired: 1 in, 3 out]
        "Green Fluorophore" <- w2932
        n2005 = property on="Get Fluorophore" class="Bool (strict)"("Val(Sgnl)"=w2932) -> ()  [unwired: 2 in, 2 out]
      }
      event User Event {
        n2006 = event-data() -> ("Boolean"=w2933:bool)  [unwired: 1 in, 3 out]
        "Red Fluorophore" <- w2933
        n2007 = property on="Get Fluorophore" class="Bool (strict)"("Val(Sgnl)"=w2933) -> ()  [unwired: 2 in, 2 out]
      }
    }
    n2008 = property on="Get Fluorophore" class="Bool (strict)"("Val(Sgnl)"="Get Fluorophore") -> ()  [unwired: 2 in, 2 out]
    n2009 = Wait (ms)(milliseconds to wait=u32 100) -> ()  [unwired: 1 out]
    n2010 = local read "Stop All"() -> (w2916:bool)
    n2011 = Or(x=w2916, y="stop") -> (x .or. y?=w2917:bool)
  }
  n2012 = timed-loop "Mouse control: trap position (AOM deflection), set confocal spot from image" {
    tunnel: [w2935] -> w207
    tunnel: w17 -> [w2934]
    timing: w129 -> [_]
    timing-out: [_] -> w128
    stop <- w2935 stop-if-true
    n2013 = node-c288() -> ()  [unwired: 2 out]
    n2014 = event shown="[0] \"Pane\": Mouse Down" {
      selector: _ -> [_ _]
      dyn-events: _ -> [_ _]
      timeout: _ -> [_ _]
      tunnel: w2934 -> [w2938 _]
      event Mouse Down {
        n2015 = event-data() -> ("Time"=w2940:u32, "Coords"=w2939:T7, "Button"=w2941:u16)  [unwired: 6 out]
        n2016 = case shown="3" w2941 {
          tunnel: w2940 -> [_ _ w3047]
          tunnel: w2939 -> [_ w2978 w3045]
          tunnel: w2938 -> [_ _ w3043]
          frame 0, Default {
          }
          frame 1 {
            n2017 = property on="APD 2" class="ImageControl"() -> ("Displayed Image Position"=w2948:cluster{"Left":i32, "Top":i32})  [unwired: 2 in, 2 out]
            n2018 = property on="APD 1" class="ImageControl"() -> ("Displayed Image Position"=w2977:cluster{"Left":i32, "Top":i32})  [unwired: 2 in, 2 out]
            n2019 = property on="Detection Laser X" class="ImageControl"() -> ("Displayed Image Position"=w2974:cluster{"Left":i32, "Top":i32})  [unwired: 2 in, 2 out]
            n2020 = property on="Detection Laser Y" class="ImageControl"() -> ("Displayed Image Position"=w2973:cluster{"Left":i32, "Top":i32})  [unwired: 2 in, 2 out]
            n2021 = property on="APD 2" class="ImageControl"() -> ("Displayed Image Size"=w2947:cluster{"Width":u32, "Height":u32})  [unwired: 2 in, 2 out]
            n2022 = property on="APD 1" class="ImageControl"() -> ("Displayed Image Size"=w2975:cluster{"Width":u32, "Height":u32})  [unwired: 2 in, 2 out]
            n2023 = property on="Detection Laser X" class="ImageControl"() -> ("Displayed Image Size"=w2976:cluster{"Width":u32, "Height":u32})  [unwired: 2 in, 2 out]
            n2024 = property on="Detection Laser Y" class="ImageControl"() -> ("Displayed Image Size"=w2972:cluster{"Width":u32, "Height":u32})  [unwired: 2 in, 2 out]
            n2025 = Unbundle By Name(w2947) -> ("Width"=w2944:u32, "Height"=w2943:u32)
            n2026 = Unbundle By Name(w2948) -> ("Left"=w2946:i32, "Top"=w2945:i32)
            n2027 = Unbundle By Name(w2975) -> ("Width"=w2969:u32, "Height"=w2968:u32)
            n2028 = Unbundle By Name(w2976) -> ("Width"=w2965:u32, "Height"=w2964:u32)
            n2029 = Unbundle By Name(w2972) -> ("Width"=w2961:u32, "Height"=w2960:u32)
            n2030 = Unbundle By Name(w2977) -> ("Left"=w2971:i32, "Top"=w2970:i32)
            n2031 = Unbundle By Name(w2974) -> ("Left"=w2967:i32, "Top"=w2966:i32)
            n2032 = Unbundle By Name(w2973) -> ("Left"=w2963:i32, "Top"=w2962:i32)
            n2033 = Bundle("Left"=w2946, "Top"=w2945, "Width"=w2944, "Height"=w2943) -> (w2942:T33)  [unwired: 1 in]